vi "Multi-Record Acquisition (Fetch One Record).vi"() -> ()   [LabVIEW 2011]
uses:
  <vilib>/userDefined/High Color/nirio_resource_hc.ctl
  <vilib>/FPGAPlugInAG/PXIe-7965R/niLvFpga_Open_PXIe-7965R.vi
  <vilib>/rvi/interface/common/dynamic/niFpgaDynamicAddResources.vi
  <vilib>/FPGAPlugInAG/Dynamic/niLvFpga_Download_Dynamic.vi
  <vilib>/FPGAPlugInAG/Dynamic/niLvFpga_Run_Dynamic.vi
  <vilib>/Utility/error.llb/Error Cluster From Error Code.vi
  <vilib>/rvi/errors/niLvFpgaAdjustHostInterfaceError.vi
  <userlib>/Host Processing Library/Windowing/LogFFT with WIndowing.vi
  <vilib>/FPGAPlugInAG/Dynamic/niLvFpga_Close_Dynamic.vi
  <vilib>/rvi/interface/nirviOpenFPGA/nirviOpenFPGA.xnode
  <userlib>/Fast OCT/Debug/Version 1/FPGA Bitfiles/Current/Acquire 2 channel data with DRAM and Frame Trigger.lvbitx
  <vilib>/rvi/interface/nirviMethod/nirviMethod.xnode
  <vilib>/rvi/interface/nirviReadWriteControl/nirviReadWriteControl.xnode
  <vilib>/rvi/interface/nirviCloseFPGA/nirviCloseFPGA.xnode
  <userlib>/FlexRIO Host Library/FlexRIO Host Library (User).lvlib
  <vilib>/rvi/interface/Simulation/niFpgaSimulationCallBeginRW.vi
  <userlib>/FlexRIO Host Library/FlexRIO Host API/Configure/Record Parameters/5772/Configure Record Parameters (5772).vi
  NiFpgaLv.dll
panel:
  out "Record Length":i32
  out "B-Scan Data":dbl[][](graph)
  in  "Device Name":T1="RIO0"
  out "RecordsFetched":i32=500
  out "Channel 0 Data":dbl[][](graph)
  out "NumSamplesAcquired":u32=406750
  in  "Stop":bool
  in  "Trigger Type":T2(ring)=enum."External Digital Trigger"
  in  "Record Count":u32=500
  in  "Pre Trig":u32=2
  in  "Post Trig":u32=1625
  out "error out":errorcluster
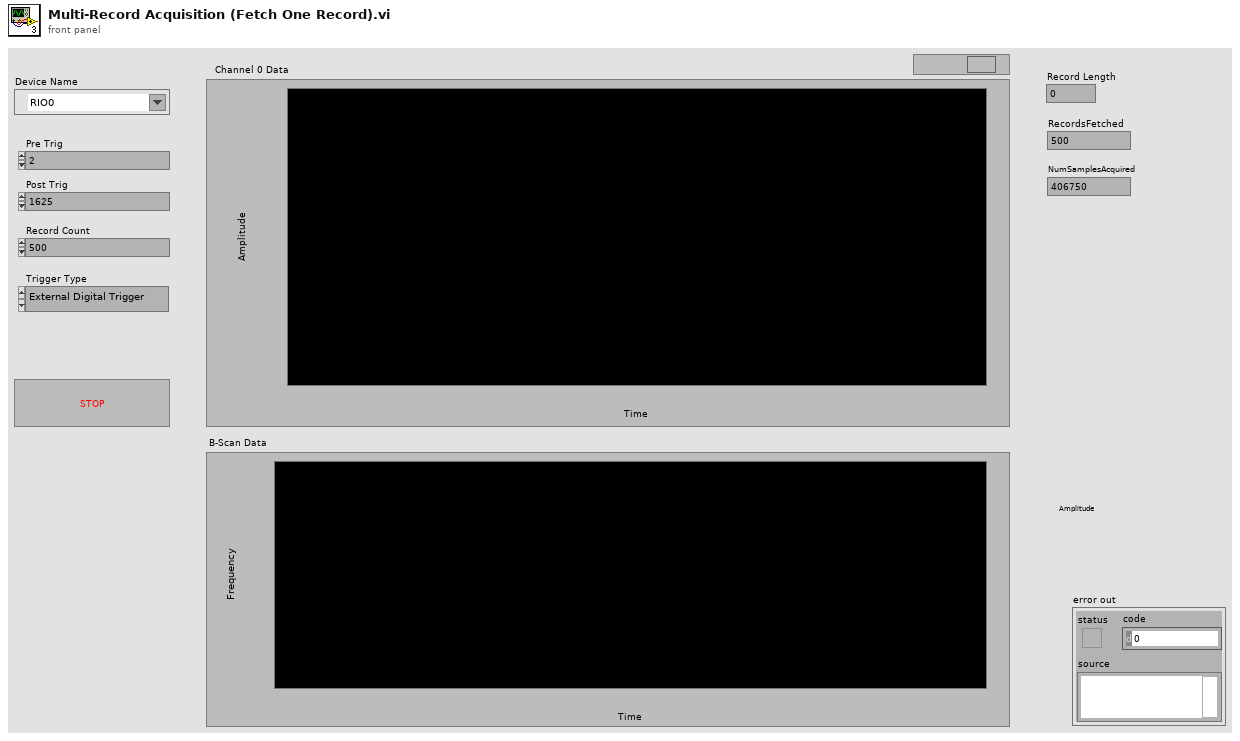
[diagram p1: front panel]
types:
  T1 = typedef "nirio_resource_hc.ctl" = tag
  T2 = enum8{"Immediate Trigger", "Software Trigger", "External Digital Trigger", "Analog Trigger"}
  T3 = cluster{"DRAM Write Ticks":u16, "DRAM Read Ticks":u16}
  T4 = cluster{"write grant time (clocks)":u16, "read grant time (clocks)":u16}
  T5 = cluster{"Load Record Parameters?":bool, "Pre Trigger Samples":u32, "Post Trigger Samples":u32, "Trigger Hold Off":u32, "Record Count":u32}
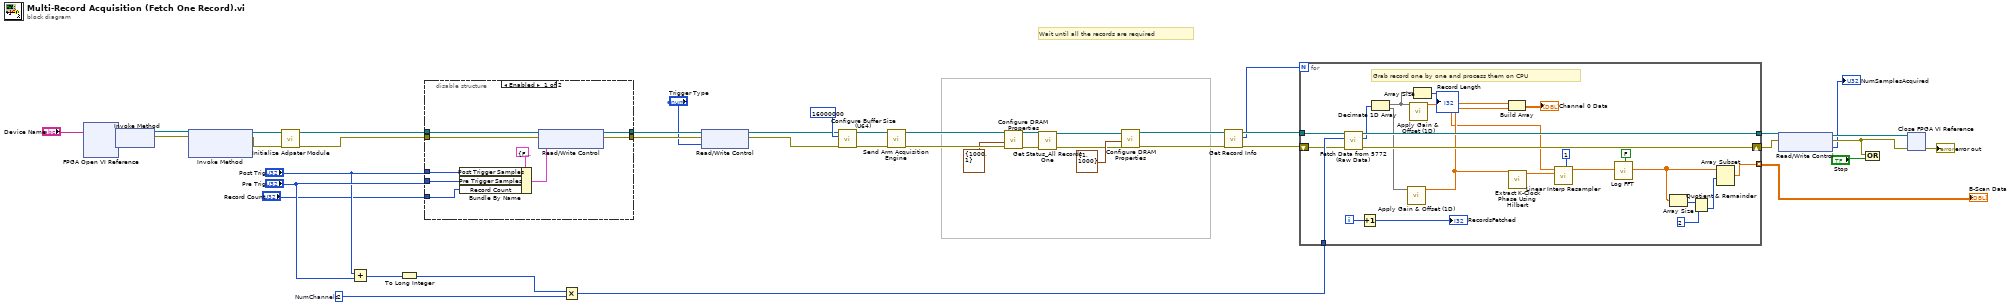
[diagram p0: block diagram]
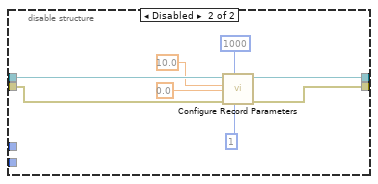
[diagram p2: hidden frame]
diagram:
  w39 = u32 2  # NumChannels
  # "Wait until all the records are required"
  n1 = xnode "FPGA Open VI Reference"("resource name"="Device Name") -> ("FPGA VI Reference Out"=w15:refnum<k20>, "error out"=w16:errorcluster)  [unwired: 1 in]
  n2 = xnode "Invoke Method"("FPGA VI Reference In"=w15, "error in"=w16) -> ("FPGA VI Reference Out"=w18:refnum<k20>, "error out"=w17:errorcluster)
  n3 = xnode "Invoke Method"("FPGA VI Reference In"=w18, "error in"=w17) -> ("FPGA VI Reference Out"=w37:refnum<k20>, "error out"=w36:errorcluster)  [unwired: 1 in]
  n4 = call <userlib>:"Initialize Adpater Module.vi"("error in"=w36, "FPGA VI Reference In"=w37) -> ("error out"=w43:errorcluster, "FPGA VI Reference Out"=w44:refnum<k20>)  [unwired: 7 in, 1 out]
  n5 = Add(x="Post Trig", y="Pre Trig") -> (x+y=w31:u32)
  n6 = To Long Integer(number=w31) -> (32bit integer=w27:i32)
  n7 = disable-structure shown="Enabled" {
    disable-tunnel: w44 -> [w54 w63]
    disable-tunnel: w43 -> [w53 w62]
    disable-tunnel: "Record Count" -> [w47 _]
    disable-tunnel: "Pre Trig" -> [w48 _]
    disable-tunnel: [w52 w60] -> w34
    disable-tunnel: [w51 w61] -> w33
    disable-tunnel: "Post Trig" -> [w49 _]
    frame Enabled {
      n8 = Bundle By Name(cluster=T5 {"Load Record Parameters?"=FALSE, "Pre Trigger Samples"=0, "Post Trigger Samples"=0, "Trigger Hold Off"=0, "Record Count"=0} ("Record Parameters"), "Post Trigger Samples"=w49, "Pre Trigger Samples"=w48, "Record Count"=w47) -> (w46:T5)
      n9 = xnode "Read/Write Control"("FPGA VI Reference In"=w54, "error in"=w53, "Record Parameters"=w46) -> ("FPGA VI Reference Out"=w52:refnum<k20>, "error out"=w51:errorcluster)
    }
    frame Disabled {
      n10 = call-poly <userlib>:"Configure Record Parameters.vi"("Record Count"=u16 1, "Record Length"=u16 1000, "error in"=w62, "% of Acquisition Hold Off Time"=0.0, "% of Pre-Trigger Samples"=10.0, "FPGA VI Reference In"=w63) -> ("error out"=w61:errorcluster, "FPGA VI Reference Out"=w60:refnum<k20>, "Actual Record Length"=w57:u16)  [unwired: 3 in]
    }
  }
  n11 = Multiply(x=w27, y=w39) -> (x*y=w38:u32)
  n12 = xnode "Read/Write Control"("FPGA VI Reference In"=w34, "error in"=w33, "Trigger Type"="Trigger Type") -> ("FPGA VI Reference Out"=w28:refnum<k20>, "error out"=w29:errorcluster)
  n13 = call <userlib>:"Configure Buffer Size (U64).vi"("error in"=w29, "Buffer Size"=u32 16000000, "FPGA VI Reference In"=w28) -> ("error out"=w21:errorcluster, "FPGA VI Reference Out"=w20:refnum<k20>)  [unwired: 7 in]
  n14 = call <userlib>:"Send Arm Acquisition Engine.vi"("error in"=w21, "FPGA VI Reference In"=w20) -> ("error out"=w12:errorcluster, "FPGA VI Reference Out"=w13:refnum<k20>)  [unwired: 8 in]
  n15 = call <userlib>:"Configure DRAM Properties.vi"("error in"=w12, "DRAM Duty Cycle"=T4 {"write grant time (clocks)"=1000, "read grant time (clocks)"=1} ("DRAM Arbiter Config"), "FPGA VI Reference In"=w13) -> ("error out"=w8:errorcluster, "FPGA VI Reference Out"=w9:refnum<k20>)  [unwired: 7 in]
  n16 = call <userlib>:"Get Status_All Records One.vi"("error in"=w8, "FPGA VI Reference In"=w9) -> ("error out"=w7:errorcluster, "FPGA VI Reference Out"=w6:refnum<k20>)  [unwired: 7 in, 1 out]
  n17 = call <userlib>:"Configure DRAM Properties.vi"("error in"=w7, "DRAM Duty Cycle"=T3 {"DRAM Write Ticks"=1, "DRAM Read Ticks"=1000}, "FPGA VI Reference In"=w6) -> ("error out"=w4:errorcluster, "FPGA VI Reference Out"=w5:refnum<k20>)  [unwired: 7 in]
  n18 = call <userlib>:"Get Record Info.vi"("error in"=w4, "FPGA VI Reference In"=w5) -> ("error out"=w3:errorcluster, "Records to Acquire"=w1:u32, "FPGA VI Reference Out"=w2:refnum<k20>)  [unwired: 7 in]
  n19 = for {
    N: w1 -> [_]
    tunnel: w38 -> [w86]
    tunnel: [w85] -> w25
    tunnel: w2 -> [w82]
    shift-right: [w84] -> w24
    shift-left: w3 -> [w81]
    tunnel: [w71] -> w14 mode=indexing
    i -> [w79]
    # "Grab record one by one and process them on CPU"
    n20 = call <userlib>:"Fetch Data from 5772 (Raw Data).vi"("error in"=w81, "Samples"=w86, "FPGA VI Reference In"=w82) -> ("error out"=w84:errorcluster, "Data Acquired"=w83:i16[], "FPGA VI Reference Out"=w85:refnum<k20>)  [unwired: 5 in, 1 out]
    n21 = Increment(x=w79) -> (x+1=→"RecordsFetched":i32)
    n22 = Decimate 1D Array(w83) -> (w65:i16[], w69:i16[])
    n23 = call <userlib>:"Apply Gain & Offset (1D).vi"("Raw Data"=w69) -> ("Scaled Data"=w68:dbl[])  [unwired: 10 in]
    n24 = call <userlib>:"Apply Gain & Offset (1D).vi"("Raw Data"=w65) -> ("Scaled Data"=w67:dbl[])  [unwired: 10 in]
    n25 = Array Size(array=w65) -> (size(s)=→"Record Length":i32)
    n26 = Build Array(w67, w68) -> (→"Channel 0 Data":dbl[][])
    n27 = call <userlib>:"Extract K-Clock Phase Using Hilbert.vi"("Input Data"=w68) -> ("Hilbert Unwrapped Phase"=w77:dbl[])  [unwired: 10 in]
    n28 = call <userlib>:"Linear Interp Resampler.vi"("interp factor"=1, "K-Data"=w77, "OCT Data"=w67) -> ("Interpolated Data"=w76:dbl[])  [unwired: 6 in, 2 out]
    n29 = call-poly <userlib>:"Log FFT.vi"("FFT Pad?"=FALSE, "FFT {X}"=w76) -> ("Log{Mag(FFT)}"=w66:dbl[])  [unwired: 9 in]
    n30 = Array Size(array=w66) -> (size(s)=w73:i32)
    n31 = Quotient & Remainder(x=w73, y=2) -> (floor(x/y)=w70:i32)  [unwired: 1 out]
    n32 = Array Subset(array=w66, index=w70) -> (w71:dbl[])  [unwired: 1 in]
  }
  "B-Scan Data" <- w14
  n33 = xnode "Read/Write Control"("FPGA VI Reference In"=w25, "error in"=w24) -> ("FPGA VI Reference Out"=w42:refnum<k20>, "error out"=w41:errorcluster, "U256s Acquired"=→"NumSamplesAcquired":u32)
  n34 = Compound Arithmetic op=OR(w41, "Stop") -> ()  [unwired: 1 out]
  n35 = xnode "Close FPGA VI Reference"("FPGA VI Reference In"=w42, "error in"=w41) -> ("error out"=→"error out":errorcluster)
